vi "01 Dryer_Performance_SM.vi"() -> ()   [LabVIEW 2012] (continued)
      }
      frame "Data: Process RMC" {
        # "FIXME: RMC calculated after power on.  Is this OK?"
        # "Process Data Steps.\nPuts the gathered data into arrays to be saved."
        n763 = local read "Init Offset Coeff"() -> (w1636:dbl)
        n764 = local read "Offset"() -> (w1637:dbl)
        n765 = Unbundle By Name(w1689) -> ("Graph Reset"=w1686:bool, "Q Element"=w1684:T10, "Enable RMC"=w1651:bool)
        n766 = call "FGV Double.vi"() -> ("Value"=w1643:dbl)  [unwired: 11 in]
        n767 = Multiply(x=w1636, y=w1643) -> (x*y=w1642:dbl)
        n768 = Add(x=w1637, y=w1642) -> (x+y=w1641:dbl)
        "Load Offset" <- w1641
        n769 = Unbundle By Name(w1684) -> ("Label Array"=w1671:string[], "Data Array"=w1668:dbl[])
        n770 = Or(x=w1686, y="Clear Graph") -> (x .or. y?=w1683:bool)
        n771 = case shown="False" w1683 {
          tunnel: [w1707 w1710] -> w1682
          tunnel: "Plot: Add Data All\nPlot: Add Data Power\nPlot: Add Data RMC" ("State(s) in Front (\"\")") -> [w1709 w1710]
          frame True {
            n772 = Concatenate Strings("Plot: Init\n" ("State(s) in Front (\"\")"), w1709) -> (w1707:string)
          }
          frame False {
          }
        }
        n773 = local read "Wet Clothing Weight"() -> (w1679:dbl)
        n774 = for {
          tunnel: w1671 -> [w1706]
          tunnel: string[] ["Weight", "Room Ambient(F)", "RDB F", "Tscale"] -> [w1705] mode=indexing
          tunnel: w1668 -> [w1704]
          tunnel: [w1702] -> w1676 mode=indexing
          n775 = Search 1D Array(1D array=w1706, element=w1705) -> (index of element=w1703:i32)  [unwired: 1 in]
          n776 = Index Array(array=w1704, index=w1703) -> (element=w1702:dbl)
        }
        n777 = local read "Init Scale Temp"() -> (w1650:dbl)
        n778 = local read "Empty Dryer Cold Weight"() -> (w1680:dbl)
        n779 = local read "BDW - Bone Dry Wt(lbs)"() -> (w1681:dbl)
        n780 = Select(t=w1641, s="Apply Load Offset", f=0.0) -> (s? t:f=w1640:dbl)
        n781 = Array To Cluster(array=w1676) -> (cluster=w1675:T32)
        n782 = Unbundle(w1675) -> ("[0]"=w1655:dbl, "[1]"=w1667:dbl, "[2]"=w1666:dbl, "[3]"=w1660:dbl)
        "Scale (LBS)" <- w1655
        "Room Ambient F" <- w1667
        "RDB F" <- w1666
        n783 = Bundle(cluster=T7 {"Measeured Weight"=0.0, "BDW - Bone Dry Wt(lbs)"=0.0, "Empty Dryer Cold Weight"=0.0, "Measured IMC"=0.0, "Tamb"=0.0, "T-RDB"=0.0, "Drum Volume"=0.0, "Load Offset"=0.0, "Temp Coeff"=0.0, "Temp Cal"=0.0, "Tscale"=0.0} ("RMC Calc Inputs 2"), "Measeured Weight"=w1655, "BDW - Bone Dry Wt(lbs)"=w1681, "Empty Dryer Cold Weight"=w1680, "Measured IMC"=w1679, "Tamb"=w1667, "T-RDB"=w1666, "Drum Volume"="Drum Volume", "Load Offset"=w1640, "Temp Coeff"="Scale Temp Coeff", "Temp Cal"=w1650, "Tscale"=w1660) -> (w1673:T7)
        "RMC Calc Inputs" <- w1673
        n784 = local read "Power On One Shot"() -> (w1654:bool)
        n785 = local read "Use Smoothing"() -> (w1644:bool)
        n786 = case shown="True" w1654 {
          tunnel: w1673 -> [_ w1701]
          tunnel: [w1692 w1700] -> w1648
          tunnel: "MA Filter Size" -> [_ w1699]
          tunnel: [_ w1698] -> w1661
          tunnel: [w1692 w1697] -> w1658
          tunnel: [_ w1696] -> w1656
          tunnel: [_ w1695] -> w1652
          tunnel: w1651 -> [_ w1694]
          tunnel: [w1692 w1693] -> w1645
          frame False {
            w1692 = 0.0 ("RMC")
          }
          frame True {
            n787 = call "MA Scale Corrections.vi"("RMC Calc Inputs"=w1701, "Enable"=w1694, "MA Filter Size"=w1699) -> ("RMC_Sm"=w1693:dbl, "RMC"=w1700:dbl, "Raw Weight"=w1698:dbl, "Corrected Weight"=w1696:dbl, "Wcomp"=w1697:dbl, "Wbouy"=w1695:dbl)  [unwired: 11 in]
          }
        }
        "Cloth Weight(est.)" <- w1656
        "Wbouy" <- w1652
        n788 = Build Array (concatenate)(w1671, "Smooth_Rmc" ("element"), "RMC" ("element"), "Raw Weight" ("element"), "Corrected Weight" ("element"), "Wcomp" ("element"), "Wbouy" ("element")) -> (w1670:string[])
        n789 = call <vilib>:"Add State(s) to Queue__jki_lib_state_machine.vi"("State(s) in Front (\"\")"=w1682, "State(s) in (\"\")"=w1691) -> ("States Out"=w1690:string)  [unwired: 13 in]
        n790 = Select(t=w1645, s=w1644, f=w1648) -> (s? t:f=→"RMC%":dbl)
        n791 = Build Array(w1645, w1648, w1661, w1656, w1658, w1652) -> (w1663:dbl[])
        n792 = Build Array (concatenate)(w1668, w1663) -> (w1669:dbl[])
        n793 = Bundle By Name(cluster=w1689, "Graph Reset"=FALSE, "Q Element.Data Array"=w1669, "Q Element.Label Array"=w1670) -> (w1688:T29)
      }
      frame "Data: Save" {
        n794 = Unbundle By Name(w1716) -> ("Init Save File"=w1719:bool, "Q Element.Label Array"=w1717:string[], "Q Element.Data Array"=w1718:dbl[], "Q Element.Date"=w1713:string)
        n795 = local read "Write to File"() -> (w1720:bool)
        n796 = case shown="True" w1720 {
          tunnel: w1719 -> [w1724 w1733]
          tunnel: w1718 -> [_ w1732]
          tunnel: w1717 -> [_ w1731]
          tunnel: [w1724 FALSE ("Init Save File")] -> w1714
          tunnel: w1713 -> [_ w1728]
          tunnel: w1712 -> [w1723 w1726]
          tunnel: [w1723 w1725] -> w1711
          frame False {
          }
          frame True {
            n797 = Build Array("Date" ("delimiter (\\t)"), w1728) -> (w1727:string[])
            n798 = local read "FileName DataLog"() -> (w1734:path)
            n799 = case shown="False" w1733 {
              tunnel: w1734 -> [w1745 w1752]
              tunnel: w1732 -> [w1744 w1751]
              tunnel: w1731 -> [w1742 _]
              tunnel: w1727 -> [w1738 _]
              tunnel: w1726 -> [w1736 w1747]
              tunnel: [w1735 w1746] -> w1725
              frame True {
                n800 = Number To Fractional String(number=w1744) -> (F-format string=w1743:string[])  [unwired: 3 in]
                n801 = Build Array(w1742, w1743) -> (w1739:string[][])
                n802 = Build Array (concatenate)(w1738, w1739) -> (w1737:string[][])
                n803 = call "Write To Spreadsheet File (string) with Error.vi"("file path (dialog if empty)"=w1745, "2D data"=w1737, "append to file? (new file:F)"=TRUE, "error in"=w1736, "delimiter (\\t)"="," ("delimiter (\\t)")) -> ("error out"=w1735:errorcluster)  [unwired: 3 in, 1 out]
              }
              frame False {
                n804 = Number To Fractional String(number=w1751) -> (F-format string=w1748:string[])  [unwired: 3 in]
                n805 = call "Write To Spreadsheet File (string) with Error.vi"("file path (dialog if empty)"=w1752, "1D data"=w1748, "append to file? (new file:F)"=TRUE, "error in"=w1747, "delimiter (\\t)"="," ("delimiter (\\t)")) -> ("error out"=w1746:errorcluster)  [unwired: 3 in, 1 out]
              }
            }
          }
        }
        n806 = call <vilib>:"Add State(s) to Queue__jki_lib_state_machine.vi"("State(s) in (\"\")"=w1722) -> ("States Out"=w1721:string)  [unwired: 14 in]
        n807 = Bundle By Name(cluster=w1716, "Init Save File"=w1714) -> (w1715:T29)
      }
      frame "------PLOT-------" {
        # "Do not put any code in this frame.\n(It is a separator no-op. You can make a copy of this frame to create a new Data frame)"
        n808 = call <vilib>:"Add State(s) to Queue__jki_lib_state_machine.vi"("State(s) in (\"\")"=w1756) -> ("States Out"=w1755:string)  [unwired: 14 in]
      }
      frame "Plot: Init" {
        w1757 = cluster{dbl[], dbl[]}[] [] ("RHS Tank TCs")
        w1763 = TRUE  # Init Save File
        w1764 = FALSE  # Graph Reset
        # "Remove Time"
        n809 = Unbundle By Name(w1762) -> ("Q Element.Label Array"=w1761:string[])
        n810 = Delete From Array(array=w1761, length=1, index=0) -> (array with subset deleted=w1760:string[])  [unwired: 1 out]
        n811 = stacked-sequence {
          tunnel: w1760 -> [w1782 _ _]
          frame #0 {
            n812 = Array Size(array=w1782) -> (size(s)=w1781:i32)
            n813 = local read "Plot Legend"() -> (w1771:T2)
            n814 = local read "Number of TCs"() -> (w1780:i32)
            n815 = Index Array(array=w1771, index=0) -> (element=w1770:T30)
            n816 = To Unsigned Long Integer(number=w1781) -> (unsigned 32bit integer=w1783:u32)
            n817 = for {
              tunnel: w1782 -> [w1786] mode=indexing
              tunnel: w1780 -> [w1793]
              tunnel: w1770 -> [w1788]
              tunnel: [w1787] -> w1769 mode=indexing
              i -> [w1794]
              n818 = Less?(x=w1794, y=w1793) -> (x < y?=w1791:bool)
              n819 = Boolean To (0,1)(Boolean=w1791) -> (0, 1=w1792:i16)
              n820 = To Unsigned Long Integer(number=w1794) -> (unsigned 32bit integer=w1795:u32)
              n821 = property on="Plot All" class="XYGraph (strict)"("Active Plot"=w1795, "Plot.Plot Name"=w1786, "Plot.YScaleIdx"=w1792) -> ("Plot.Plot Color"=w1789:u32)  [unwired: 2 in, 2 out]
              n822 = Bundle By Name(cluster=w1788, "OnOff"=TRUE ("Boolean"), "Color Box"=w1789, "Title"=w1786) -> (w1787:T30)
            }
            n823 = property on="Plot All" class="XYGraph (strict)"("XScale.NameLbl.Text"="Time" ("X Scale.Name Label.Text"), "ActYScl"=1 ("Active Y Scale"), "YScale.NameLbl.Text"="Temperature °F" ("X Scale Label"), "YScale.Minimum"=50.0 ("Y Scale.Range:Minimum"), "YScale.Maximum"=200.0 ("Y Scale.Range:Maximum"), "ActYScl"=0 ("Active Y Scale"), "YScale.NameLbl.Text"="kWatts, lbs.,V,A" ("Y Scale Label Right"), "YScale.Minimum"=0.0 ("Ymin Right"), "YScale.Maximum"=250.0 ("Y Scale.Range:Maximum"), "LegNumRows"=w1783) -> ()  [unwired: 2 in, 2 out]
            n824 = local write "Plot Legend"(w1769) -> ()
          }
          frame #1 {
            w1805 = string[] ["Irms:Element 1", "Irms:Element 2", "P:Sigma"]
            n825 = control-ref of="Plot Power"() -> (w1796:refnum<vi>)
            n826 = for {
              tunnel: w1805 -> [w1816] mode=indexing
              tunnel: 2 ("y") -> [w1811]
              tunnel: w1796 -> [w1810]
              i -> [w1814]
              n827 = Greater Or Equal?(x=w1814, y=w1811) -> (x >= y?=w1812:bool)
              n828 = Boolean To (0,1)(Boolean=w1812) -> (0, 1=w1813:i16)
              n829 = To Unsigned Long Integer(number=w1814) -> (unsigned 32bit integer=w1815:u32)
              n830 = property on="Property Node" class="XYGraph (strict)"(reference=w1810, "Active Plot"=w1815, "Plot.Plot Name"=w1816, "Plot.YScaleIdx"=w1813) -> ()  [unwired: 1 in, 2 out]
            }
            n831 = Array Size(array=w1805) -> (size(s)=w1808:i32)
            n832 = To Unsigned Long Integer(number=w1808) -> (unsigned 32bit integer=w1806:u32)
            n833 = property on="Property Node" class="XYGraph (strict)"(reference=w1796, "XScale.NameLbl.Text"="Time" ("X Scale.Name Label.Text"), "ActYScl"=1 ("Active Y Scale"), "YScale.NameLbl.Text"="Watts" ("Y Scale.Name Label.Text"), "YScale.Minimum"=0.0 ("Y Scale.Range:Minimum"), "YScale.Maximum"=5000.0 ("Y Scale.Range:Maximum"), "ActYScl"=0 ("Active Y Scale"), "YScale.NameLbl.Text"="Current(Amps)" ("Y Scale.Name Label.Text"), "YScale.Minimum"=0.0 ("Y Scale.Range:Minimum"), "YScale.Maximum"=32.0 ("Y Scale.Range:Maximum"), "LegNumRows"=w1806) -> ()  [unwired: 1 in, 2 out]
          }
          frame #2 {
            w1824 = string[] ["RAW Weight", "RMC"]
            n834 = control-ref of="Plot RMC"() -> (w1817:refnum<vi>)
            n835 = Array Size(array=w1824) -> (size(s)=w1827:i32)
            n836 = for {
              tunnel: w1824 -> [w1834] mode=indexing
              tunnel: w1817 -> [w1829]
              i -> [w1832]
              n837 = Equal To 0?(x=w1832) -> (x = 0?=w1830:bool)
              n838 = Boolean To (0,1)(Boolean=w1830) -> (0, 1=w1831:i16)
              n839 = To Unsigned Long Integer(number=w1832) -> (unsigned 32bit integer=w1833:u32)
              n840 = property on="Property Node" class="XYGraph (strict)"(reference=w1829, "Active Plot"=w1833, "Plot.Plot Name"=w1834, "Plot.YScaleIdx"=w1831) -> ()  [unwired: 1 in, 2 out]
            }
            n841 = To Unsigned Long Integer(number=w1827) -> (unsigned 32bit integer=w1825:u32)
            n842 = property on="Property Node" class="XYGraph (strict)"(reference=w1817, "XScale.NameLbl.Text"="Time" ("X Scale.Name Label.Text"), "ActYScl"=1 ("Active Y Scale"), "YScale.NameLbl.Text"="LBS" ("Y Scale.Name Label.Text"), "AutoscaleDelay"=sgl 0.0 ("Autoscale Delay"), "ActYScl"=0 ("Active Y Scale"), "YScale.NameLbl.Text"="RMC" ("Y Scale.Name Label.Text"), "YScale.Minimum"=0.0 ("Y Scale.Range:Minimum"), "YScale.Maximum"=100.0 ("Y Scale.Range:Maximum"), "LegNumRows"=w1825) -> ()  [unwired: 1 in, 2 out]
          }
        }
        n843 = Bundle By Name(cluster=w1762, "Graph Reset"=w1764, "Init Save File"=w1763) -> (w1765:T29)
        n844 = local write "Plot All"(w1757) -> ()
        n845 = local write "Plot Power"(w1757) -> ()
        n846 = local write "Plot RMC"(w1757) -> ()
        n847 = call <vilib>:"Add State(s) to Queue__jki_lib_state_machine.vi"("State(s) in (\"\")"=w1768) -> ("States Out"=w1767:string)  [unwired: 14 in]
      }
      frame "Plot: Add Data All" {
        # "Add Current Sample to Data Array"
        # "First Element Assumed to be Time."
        n848 = Unbundle By Name(w1854) -> ("Time Array"=w1853:dbl[], "Q Element.Data Array"=w1848:dbl[], "Data Array"=w1856:dbl[][])
        n849 = case shown="True" "None" {
          selector: "None" -> [w1868 _]
          tunnel: "Plot Legend" -> [w1869 w1872]
          tunnel: [w1869 w1871] -> w1839
          tunnel: [w1868 w1870] -> w1836
          frame False {
          }
          frame True {
            n850 = for {
              tunnel: w1872 -> [w1875] mode=indexing
              tunnel: [w1874] -> w1871 mode=indexing
              tunnel: [w1873] -> w1870
              w1873 = FALSE ("OnOff")
              n851 = Bundle By Name(cluster=w1875, "OnOff"=w1873) -> (w1874:T30)
            }
          }
        }
        n852 = local write "None"(w1836) -> ()
        n853 = case shown="True" "All" {
          tunnel: w1839 -> [w1861 w1864]
          tunnel: [w1861 w1863] -> w1837
          tunnel: [FALSE ("OnOff") FALSE ("OnOff")] -> w1835
          frame False {
          }
          frame True {
            n854 = for {
              tunnel: w1864 -> [w1867] mode=indexing
              tunnel: [w1866] -> w1863 mode=indexing
              n855 = Bundle By Name(cluster=w1867, "OnOff"=TRUE) -> (w1866:T30)
            }
          }
        }
        n856 = Delete From Array(array=w1848, length=1, index=0) -> (deleted portion=w1846:dbl[], array with subset deleted=w1847:dbl[])
        n857 = Transpose 2D Array(2D array=w1856) -> (transposed array=w1851:dbl[][])
        n858 = Build Array (concatenate)(w1853, w1846) -> (w1849:dbl[])
        n859 = Build Array (concatenate)(w1851, w1847) -> (w1852:dbl[][])
        n860 = Transpose 2D Array(2D array=w1852) -> (transposed array=w1850:dbl[][])
        n861 = control-ref of="Plot All"() -> (w1842:refnum<vi>)
        n862 = local write "Plot Legend"(w1837) -> ()
        n863 = local write "All"(w1835) -> ()
        n864 = for {
          tunnel: w1849 -> [w1882]
          tunnel: [w1881] -> w1843 mode=indexing
          tunnel: w1850 -> [w1880] mode=indexing
          tunnel: w1842 -> [w1879]
          tunnel: w1837 -> [w1877] mode=indexing
          i -> [w1878]
          n865 = Unbundle By Name(w1877) -> ("OnOff"=w1876:bool)
          n866 = Bundle(w1882, w1880) -> (w1881:cluster{dbl[], dbl[]})  [unwired: 1 out]
          n867 = property on="Property Node" class="XYGraph (strict)"(reference=w1879, "Active Plot"=w1878, "Plot.Visible?"=w1876) -> ()  [unwired: 1 in, 2 out]
        }
        "Plot All" <- w1843
        n868 = call <vilib>:"Add State(s) to Queue__jki_lib_state_machine.vi"("State(s) in (\"\")"=w1859) -> ("States Out"=w1858:string)  [unwired: 14 in]
        n869 = Bundle By Name(cluster=w1854, "Time Array"=w1849, "Data Array"=w1850) -> (w1855:T29)
      }
      frame "Plot: Add Data Power" {
        n870 = Unbundle By Name(w1900) -> ("Q Element.Label Array"=w1899:string[], "Time Array"=w1901:dbl[], "Data Array"=w1891:dbl[][])
        n871 = for {
          tunnel: w1899 -> [w1908]
          tunnel: string[] ["Irms:Element 1", "Irms:Element 2", "P:Sigma"] -> [w1907] mode=indexing
          tunnel: [w1906] -> w1898 mode=indexing
          n872 = Search 1D Array(1D array=w1908, element=w1907) -> (index of element=w1906:i32)  [unwired: 1 in]
        }
        n873 = Index Array(array=w1898, index #1=0 ("index"), index #2=1 ("index"), index #3=2 ("index")) -> (element #1=w1894:i32, element #2=w1893:i32, element #3=w1892:i32)
        n874 = Decrement(x=w1893) -> (x-1=w1884:i32)
        n875 = Decrement(x=w1894) -> (x-1=w1885:i32)
        n876 = Decrement(x=w1892) -> (x-1=w1883:i32)
        n877 = Index Array(array=w1891, index (row)=w1885) -> (element=w1890:dbl[])  [unwired: 1 in]
        n878 = Index Array(array=w1891, index (row)=w1884) -> (element=w1889:dbl[])  [unwired: 1 in]
        n879 = Index Array(array=w1891, index (row)=w1883) -> (element=w1888:dbl[])  [unwired: 1 in]
        n880 = Build Array(w1890, w1889, w1888) -> (w1887:dbl[][])
        n881 = for {
          tunnel: w1901 -> [w1911]
          tunnel: [w1910] -> w1902 mode=indexing
          tunnel: w1887 -> [w1909] mode=indexing
          n882 = Bundle("Time Array"=w1911, w1909) -> (w1910:cluster{"Time Array":dbl[], dbl[]})  [unwired: 1 out]
        }
        "Plot Power" <- w1902
        n883 = call <vilib>:"Add State(s) to Queue__jki_lib_state_machine.vi"("State(s) in (\"\")"=w1905) -> ("States Out"=w1904:string)  [unwired: 14 in]
      }
      frame "Plot: Add Data RMC" {
        # "Is the dry time and exponential?"
        n884 = Unbundle By Name(w1942) -> ("Q Element.Label Array"=w1941:string[], "Time Array"=w1931:dbl[], "Data Array"=w1912:dbl[][])
        n885 = local read "Debug Mode"() -> (w1920:bool)
        n886 = Select(t="RMC", s=w1920, f="Smooth_Rmc") -> (s? t:f=w1917:string)
        n887 = Build Array("Weight", w1917) -> (w1916:string[])
        n888 = for {
          tunnel: w1941 -> [w1949]
          tunnel: w1916 -> [w1948] mode=indexing
          tunnel: [w1947] -> w1940 mode=indexing
          n889 = Search 1D Array(1D array=w1949, element=w1948) -> (index of element=w1947:i32)  [unwired: 1 in]
        }
        n890 = local read "BDW - Bone Dry Wt(lbs)"() -> (w1925:dbl)
        n891 = local read "RMC Limit"() -> (w1929:dbl)
        n892 = Index Array(array=w1940, index #1=0 ("index"), index #2=1 ("index"), index #3=2 ("index")) -> (element #1=w1937:i32, element #2=w1936:i32, element #3=w1914:i32)
        n893 = local read "Wet Clothing Weight"() -> (w1930:dbl)
        n894 = Decrement(x=w1936) -> (x-1=w1932:i32)
        n895 = Decrement(x=w1937) -> (x-1=w1933:i32)
        n896 = Decrement(x=w1914) -> (x-1=w1913:i32)
        n897 = Index Array(array=w1912, index (row)=w1933) -> (element=w1923:dbl[])  [unwired: 1 in]
        n898 = Index Array(array=w1912, index (row)=w1932) -> (element=w1935:dbl[])  [unwired: 1 in]
        n899 = Divide(x=w1929, y=100.0) -> (x/y=w1927:dbl)
        n900 = Index Array(array=w1912, index (row)=w1913) -> ()  [unwired: 1 in, 1 out]
        n901 = Multiply(x=w1925, y=w1927) -> (x*y=w1926:dbl)
        n902 = Build Array(w1923, w1935) -> (w1934:dbl[][])
        n903 = Add(x=w1925, y=w1926) -> (x+y=w1924:dbl)
        n904 = for {
          tunnel: w1931 -> [w1952]
          tunnel: [w1951] -> w1943 mode=indexing
          tunnel: w1934 -> [w1950] mode=indexing
          n905 = Bundle("Time Array"=w1952, w1950) -> (w1951:cluster{"Time Array":dbl[], dbl[]})  [unwired: 1 out]
        }
        "Plot RMC" <- w1943
        n906 = call "Estimate Exp Completion time.vi"("IMC Weight"=w1930, "Completion Weight"=w1924, "Time Values"=w1931, "Weight Values"=w1923) -> ("Completion Time Estimate"=→"Experimental Completion Time Estimate":dbl)  [unwired: 9 in, 2 out]
        n907 = call <vilib>:"Add State(s) to Queue__jki_lib_state_machine.vi"("State(s) in (\"\")"=w1946) -> ("States Out"=w1945:string)  [unwired: 14 in]
      }
      frame "-------FINALIZE------ " {
        n908 = call <vilib>:"Add State(s) to Queue__jki_lib_state_machine.vi"("State(s) in (\"\")"=w1956) -> ("States Out"=w1955:string)  [unwired: 14 in]
      }
      frame "Finalize Sequence" {
        n909 = local read "FileName DataLog"() -> (w1960:path)
        n910 = local read "Write to File"() -> (w1959:bool)
        n911 = call <vilib>:"Check if File or Folder Exists.vi"("path"=w1960) -> ("file or folder exists?"=w1958:bool)  [unwired: 8 in, 2 out]
        n912 = And(x=w1958, y=w1959) -> (x .and. y?=w1957:bool)
        n913 = case shown="True" w1957 {
          tunnel: [_ "Finalize DataLog\nFinalize Write DOE Data\nFinalize Move and Lock Files\nFinalize Zip Files" ("State(s) in Front (\"\")")] -> w1961
          frame False {
          }
          frame True {
          }
        }
        n914 = call <vilib>:"Add State(s) to Queue__jki_lib_state_machine.vi"("State(s) in Front (\"\")"=w1961, "State(s) in (\"\")"=w1965) -> ("States Out"=w1964:string)  [unwired: 13 in]
      }
      frame "Finalize DataLog" {
        w1971 = 60.0  # s/min
        # "RMC OK?"
        n915 = case shown="True" "Auto Scale Reading" {
          tunnel: [w2028 w2035] -> w2013
          tunnel: [w2026 w2033] -> w1974
          frame False {
            n916 = flat-sequence {
              tunnel: [w2030] -> w2027
              tunnel: [w2032] -> w2028
              tunnel: w2027 -> [w2032]
              tunnel: [w2031] -> w2026
              frame #0 {
                n917 = call "Panel Get Final Weight.vi"("Init value(\"\")"="0." ("Init value(\"\")")) -> ("Final Load  Weight Out"=w2030:string)  [unwired: 14 in]
              }
              frame #1 {
                n918 = call "E-Time.vi"() -> ("Elapsed Time (sec)"=w2031:dbl)  [unwired: 9 in, 2 out]
              }
            }
          }
          frame True {
            n919 = flat-sequence {
              tunnel: [w2037] -> w2034
              tunnel: [w2039] -> w2035
              tunnel: w2034 -> [w2039]
              tunnel: [w2038] -> w2033
              frame #0 {
                n920 = local read "Scale Com Port"() -> (w2036:refnum<visa-resource-name>)
                n921 = call "Panel Scale Reading Percision.vi"("VISA resource name"=w2036) -> ("read buffer"=w2037:string)  [unwired: 14 in]
              }
              frame #1 {
                n922 = call "E-Time.vi"() -> ("Elapsed Time (sec)"=w2038:dbl)  [unwired: 9 in, 2 out]
              }
            }
          }
        }
        n923 = Unbundle By Name(w2017) -> ("Q Element.Label Array"=w1987:string[], "Q Element.Data Array"=w1988:dbl[])
        n924 = local read "FileName DataLog"() -> (w1977:path)
        n925 = call "Log String to Spreadsheet.vi"("String"="Stopped", "error in (no error)"=w2018, "FileName"=w1977) -> ("error out"=w2015:errorcluster)  [unwired: 8 in]
        n926 = for {
          tunnel: w1987 -> [w2025]
          tunnel: string[] ["Time", "Gas Feedback", "Wp:Sigma"] -> [w2024] mode=indexing
          tunnel: w1988 -> [w2023]
          tunnel: [w2021] -> w1989 mode=indexing
          n927 = Search 1D Array(1D array=w2025, element=w2024) -> (index of element=w2022:i32)  [unwired: 1 in]
          n928 = Index Array(array=w2023, index=w2022) -> (element=w2021:dbl)
        }
        n929 = Fract/Exp String To Number(string=w2013) -> (number=w1991:dbl)  [unwired: 3 in, 1 out]
        n930 = local read "Use Dry Gas Meter?"() -> (w1984:bool)
        n931 = Concatenate Strings("Final Weight:, " ("String"), w2013) -> (w2007:string)
        n932 = local read "Enable RMC Limit"() -> (w1975:bool)
        n933 = local read "Power On One Shot"() -> (w2000:bool)
        n934 = call "Log String to Spreadsheet.vi"("String"=w2007, "error in (no error)"=w2015, "FileName"=w1977) -> ("error out"=w1979:errorcluster)  [unwired: 8 in]
        n935 = Array To Cluster(array=w1989) -> (cluster=w1990:cluster{"[0]":dbl, "[1]":dbl, "[2]":dbl})
        n936 = Unbundle(w1990) -> ("[0]"=w1973:dbl, "[1]"=w1981:dbl, "[2]"=w1980:dbl)
        n937 = Subtract(x=w1974, y=w1973) -> (x-y=w1972:dbl)
        n938 = Divide(x=w1972, y=w1971) -> (x/y=w1970:dbl)
        n939 = Number To Fractional String(number=w1970) -> (F-format string=w1969:string)  [unwired: 3 in]
        n940 = And(x=w1975, y=w2000) -> (x .and. y?=w2001:bool)
        n941 = Concatenate Strings("FMC DELAY (min):," ("String"), w1969) -> (w1968:string)
        n942 = call "Log String to Spreadsheet.vi"("String"=w1968, "error in (no error)"=w1979, "FileName"=w1977) -> ("error out"=w1978:errorcluster)  [unwired: 8 in]
        n943 = case shown="True" w2001 {
          tunnel: [TRUE w2041] -> w1999
          frame False {
          }
          frame True {
            n944 = local read "RMC Limit"() -> (w2042:dbl)
            n945 = local read "RMC%"() -> (w2043:dbl)
            n946 = Greater?(x=w2042, y=w2043) -> (0:w2041:bool)
          }
        }
        n947 = local read "BDW - Bone Dry Wt(lbs)"() -> (w2012:dbl)
        n948 = Select(t=w1981, s=w1984, f=0.0) -> (s? t:f=w1983:dbl)
        n949 = local read "End Msg"() -> (w2004:string)
        n950 = call "Log String to Spreadsheet.vi"("String"=w2004, "error in (no error)"=w1978, "FileName"=w1977) -> ()  [unwired: 8 in, 1 out]
        n951 = Divide(x=w1991, y=w2012) -> (x/y=w2011:dbl)
        n952 = call "Worksheet DOE Audit.vi"() -> ("DOE Data Out"=w1993:T23)  [unwired: 8 in, 2 out]
        n953 = Bundle By Name(cluster=w1993, "End Time(s)"=w1973, "Final Wt"=w1991, "Gas Vol Fin"=w1983, "Elect Energy End"=w1980) -> (w1992:T23)
        n954 = Decrement(x=w2011) -> (x-1=w2008:dbl)
        n955 = Search and Replace String(replace all?=TRUE ("replace all? (F)"), input string=w2004, search string=",") -> (result string=w2002:string)  [unwired: 5 in, 3 out]
        n956 = Number To Fractional String(number=w2008) -> (F-format string=w2010:string)  [unwired: 3 in]
        n957 = local read "2015?"() -> (w1967:bool)
        n958 = call "Worksheet DOE Audit.vi"("Add?"=TRUE, "DOE Data"=w1992, "2015?"=w1967) -> ()  [unwired: 5 in, 3 out]
        n959 = Concatenate Strings(w2002, "\r", "Final RMC:" ("String"), w2010) -> (w1998:string)
        n960 = call <vilib>:"Add State(s) to Queue__jki_lib_state_machine.vi"("State(s) in (\"\")"=w2020) -> ("States Out"=w2019:string)  [unwired: 14 in]
        n961 = Append True/False String(1:w1999, 2:". RMC Limit Not Reached." ("false string"), 3:"" ("true string"), 4:w1998) -> (0:→"Final User Message":string)
      }
      frame "Finalize Write DOE Data" {
        n962 = local read "FileName DataLog"() -> (w2045:path)
        n963 = call <vilib>:"Check if File or Folder Exists.vi"("path"=w2045) -> ("file or folder exists?"=w2046:bool)  [unwired: 8 in, 2 out]
        n964 = local read "2015?"() -> (w2044:bool)
        n965 = case shown="True" w2046 {
          tunnel: w2045 -> [_ w2052]
          tunnel: w2044 -> [_ w2051]
          frame False {
          }
          frame True {
            n966 = case shown="True" w2051 {
              tunnel: w2052 -> [w2063 w2069]
              frame False {
                n967 = Strip Path(path=w2063) -> (name=w2059:string)  [unwired: 1 out]
                n968 = Search and Replace String(input string=w2059, search string=".tmp", replace string="_OUT.txt" ("replace string (\"\")")) -> (result string=w2061:string)  [unwired: 5 in, 3 out]
                n969 = global read "Global Test Variables DPT.vi" "Globals for Dryer Performance Test"() -> (w2058:T9)
                n970 = Unbundle By Name(w2058) -> ("Directories.Data Backup Directory"=w2057:path)
                n971 = local read "2015?"() -> (w2055:bool)
                n972 = call "Worksheet DOE Audit.vi"("Write Form"=TRUE ("Add?"), "2015?"=w2055) -> ("String"=w2053:string)  [unwired: 6 in, 2 out]
                n973 = Build Path(base path=w2057, name or relative path=w2061) -> (appended path=w2054:path)
                "DOE Filename" <- w2054
                n974 = call "File Write with Filename.vi"("Path"=w2054, "text"=w2053) -> ()  [unwired: 12 in, 2 out]
                n975 = One Button Dialog(message=w2053) -> ()  [unwired: 1 in, 1 out]
              }
              frame True {
                n976 = Strip Path(path=w2069) -> (name=w2074:string)  [unwired: 1 out]
                n977 = Search and Replace String(input string=w2074, search string=".tmp", replace string="_OUT.csv" ("replace string (\"\")")) -> (result string=w2076:string)  [unwired: 5 in, 3 out]
                n978 = global read "Global Test Variables DPT.vi" "Globals for Dryer Performance Test"() -> (w2073:T9)
                n979 = Unbundle By Name(w2073) -> ("Directories.Data Backup Directory"=w2072:path)
                n980 = local read "Low Power Switch"() -> (w2065:bool)
                n981 = local read "2015?"() -> (w2070:bool)
                n982 = call "Worksheet DOE Audit.vi"("Write Form"=TRUE ("Add?"), "Low Power\nSwitch"=w2065, "2015?"=w2070) -> ("String"=w2064:string, "2015 array"=w2066:string[][])  [unwired: 5 in, 1 out]
                n983 = Build Path(base path=w2072, name or relative path=w2076) -> (appended path=w2068:path)
                n984 = local write "DOE Filename"(w2068) -> ()
                n985 = call-poly <vilib>:"Write To Spreadsheet File.vi"("delimiter (\\t)"="," ("delimiter (\\t)"), "2D data"=w2066, "file path (dialog if empty)"=w2068) -> ()  [unwired: 5 in, 1 out]
                n986 = One Button Dialog(message=w2064) -> ()  [unwired: 1 in, 1 out]
              }
            }
          }
        }
        n987 = call <vilib>:"Add State(s) to Queue__jki_lib_state_machine.vi"("State(s) in (\"\")"=w2050) -> ("States Out"=w2049:string)  [unwired: 14 in]
      }
      frame "Finalize Move and Lock Files" {
        n988 = local read "FileName DataLog"() -> (w2078:path)
        n989 = stacked-sequence {
          tunnel: w2078 -> [w2086 _ _ w2120]
          frame #0 {
            # "DC Voltages"
            n990 = Strip Path(path=w2086) -> (name=w2084:string)  [unwired: 1 out]
            n991 = Match Pattern(string=w2084, regular expression=".tmp" ("search string")) -> (before substring=→"Filename Prefix String":string)  [unwired: 1 in, 3 out]
          }
          frame #1 {
            # "DC Voltages"
            n992 = local read "Stream DC to File?"() -> (w2087:bool)
            n993 = case shown="True" w2087 {
              frame False {
              }
              frame True {
                n994 = global read "Global Test Variables DPT.vi" "Globals for Dryer Performance Test"() -> (w2096:T9)
                n995 = local read "Filename Prefix String"() -> (w2089:string)
                n996 = Unbundle By Name(w2096) -> ("Directories.Data Backup Directory"=w2095:path)
                n997 = local read "DC Voltages Filename"() -> (w2093:path)
                n998 = Concatenate Strings(w2089, "_DC_VOLTAGES.csv" ("search string")) -> (w2088:string)
                n999 = Build Path(base path=w2095, name or relative path=w2088) -> (appended path=w2092:path)
                n1000 = Copy(10:w2092, 11:w2093) -> (3:w2091:path)  [unwired: 3 in, 2 out]
                n1001 = local write "DC Voltages Filename"(w2091) -> ()
                n1002 = Set Permissions(7:i16 0 ("permissions"), 11:w2091) -> (0:w2097:errorcluster)  [unwired: 3 in, 1 out]
                n1003 = Merge Errors(w2097) -> ()  [unwired: 1 out]
              }
            }
          }
          frame #2 {
            n1004 = local read "Nufi?"() -> (w2098:bool)
            n1005 = case shown="False" w2098 {
              frame False {
              }
              frame True {
                n1006 = global read "Global Test Variables DPT.vi" "Globals for Dryer Performance Test"() -> (w2107:T9)
                n1007 = while {
                  tunnel: [w2111] -> w2105
                  stop <- w2111 stop-if-true
                  n1008 = local read "End4_Nufi"() -> (w2111:bool)
                  n1009 = case shown="False" w2111 {
                    frame False {
                      n1010 = Wait (ms)(milliseconds to wait=u32 250) -> ()  [unwired: 1 out]
                    }
                    frame True {
                    }
                  }
                }
                n1011 = local read "Filename Prefix String"() -> (w2100:string)
                n1012 = Unbundle By Name(w2107) -> ("Directories.Data Backup Directory"=w2106:path)
                n1013 = Concatenate Strings(w2100, "_NUFI_DEBUG.csv" ("search string")) -> (w2099:string)
                n1014 = flat-sequence {
                  tunnel: [w2110] -> w2103
                  tunnel: w2105 -> [_]
                  frame #0 {
                    n1015 = local read "Nufi Data File Path"() -> (w2110:path)
                  }
                }
                n1016 = Build Path(base path=w2106, name or relative path=w2099) -> (appended path=w2104:path)
                n1017 = Copy(10:w2104, 11:w2103) -> (3:w2102:path)  [unwired: 3 in, 2 out]
                n1018 = Set Permissions(7:i16 0 ("permissions"), 11:w2102) -> (0:w2108:errorcluster)  [unwired: 3 in, 1 out]
                n1019 = local write "Nufi Data File Path"(w2102) -> ()
                n1020 = Merge Errors(w2108) -> ()  [unwired: 1 out]
              }
            }
          }
          frame #3 {
            # "DATA LOG"
            n1021 = global read "Global Test Variables DPT.vi" "Globals for Dryer Performance Test"() -> (w2117:T9)
            n1022 = local read "Filename Prefix String"() -> (w2114:string)
            n1023 = Unbundle By Name(w2117) -> ("Directories.Data Backup Directory"=w2116:path)
            n1024 = Concatenate Strings(w2114, ".csv" ("search string")) -> (w2113:string)
            n1025 = Build Path(base path=w2116, name or relative path=w2113) -> (appended path=w2119:path)
            n1026 = Copy(10:w2119, 11:w2120) -> (3:w2118:path)  [unwired: 3 in, 2 out]
            n1027 = local write "FileName DataLog"(w2118) -> ()
          }
        }
        n1028 = call <vilib>:"Add State(s) to Queue__jki_lib_state_machine.vi"("State(s) in (\"\")"=w2082) -> ("States Out"=w2081:string)  [unwired: 14 in]
      }
      frame "Finalize Zip Files" {
        n1029 = local read "FileName DataLog"() -> (w2127:path)
        n1030 = global read "Global Test Variables DPT.vi" "Globals for Dryer Performance Test"() -> (w2149:T9)
        n1031 = while {
          tunnel: [w2156] -> w2123
          stop <- w2157 stop-if-true
          n1032 = local read "Nufi Data File Path"() -> (w2156:path)
          n1033 = local read "End4_Nufi"() -> (w2157:bool)
          n1034 = Wait (ms)(milliseconds to wait=u32 150) -> ()  [unwired: 1 out]
        }
        n1035 = local read "Stream DC to File?"() -> (w2150:bool)
        n1036 = Unbundle By Name(w2149) -> ("Directories.Save File Directory"=w2148:path, "Directories.Library Directory"=w2135:path, "Directories.Data Backup Dir Fail"=w2134:path, "Directories.Lab Directory"=w2133:path)
        n1037 = call <vilib>:"Three Button Dialog.vi"("Allow user to close window? (TRUE)"=FALSE, "Right Button Text (\"Cancel\")"="Lab Eval" ("Right Button Text (\"Cancel\")"), "Center Button Text (\"No\")"="Fail" ("F button name (\"Cancel\")"), "Left Button Text (\"Yes\")"="Pass" ("T button name (\"OK\")"), "message"="Final Test Result.  \"Pass\" will log data to the backup server.  \"Fail\" will copy files to another location.") -> ("Which Button?"=w2137:T33)  [unwired: 6 in]
        n1038 = case shown="True" w2150 {
          tunnel: [_ w2186] -> w2126
          frame False {
          }
          frame True {
            n1039 = local read "DC Voltages Filename"() -> (w2186:path)
          }
        }
        n1040 = case shown="\"Center Button\"" w2137 {
          tunnel: [w2175 w2180 w2185] -> w2136
          tunnel: w2135 -> [w2175 _ _]
          tunnel: w2134 -> [_ w2180 _]
          tunnel: w2133 -> [_ _ w2185]
          tunnel: ["Result: Pass" ("T button name (\"OK\")") w2177 w2182] -> w2132
          tunnel: [TRUE FALSE FALSE] -> w2128
          frame "Left Button", Default {
          }
          frame "Center Button" {
            n1041 = call "Prompt User for Input"() -> ("Reason for Failure"=w2178:string)  [unwired: 17 in, 2 out]
            n1042 = Concatenate Strings("Result: Fail - ", w2178) -> (w2177:string)
          }
          frame "Right Button" {
            n1043 = call "Prompt User for Input2"() -> ("Eval Description"=w2183:string)  [unwired: 17 in, 2 out]
            n1044 = Concatenate Strings("Result:  Eval -", w2183) -> (w2182:string)
          }
        }
        n1045 = call "Log String to Spreadsheet.vi"("String"=w2132, "error in (no error)"=w2124, "FileName"=w2127) -> ("error out"=w2130:errorcluster)  [unwired: 8 in]
        n1046 = local read "Filename Prefix String"() -> (w2145:string)
        n1047 = Set Permissions(7:i16 0 ("permissions"), 8:w2130, 11:w2127) -> (0:w2122:errorcluster)  [unwired: 2 in, 1 out]
        n1048 = case shown="False" w2128 {
          tunnel: w2127 -> [w2164 w2169]
          tunnel: w2126 -> [w2165 w2171]
          tunnel: w2123 -> [w2160 w2170]
          tunnel: [w2162 w2168] -> w2125
          tunnel: w2122 -> [w2159 w2167]
          tunnel: [w2158 w2167] -> w2121
          frame True {
            n1049 = call <vilib>:"Check if File or Folder Exists.vi"("path"=w2160) -> ("file or folder exists?"=w2161:bool)  [unwired: 8 in, 2 out]
            n1050 = local read "DOE Filename"() -> (w2166:path)
            n1051 = call "Parser Dryer Performance.vi"("error in"=w2159, "Process Debug?"=w2161, "log file path in"=w2164, "debug log path in"=w2160) -> ("error out"=w2158:errorcluster, "new file path out"=w2163:path)  [unwired: 6 in]
            n1052 = Build Array(w2166, w2164, w2165, w2160, w2163) -> (w2162:path[])
          }
          frame False {
            n1053 = local read "DOE Filename"() -> (w2172:path)
            n1054 = Build Array(w2172, w2169, w2171, w2170) -> (w2168:path[])
          }
        }
        n1055 = Concatenate Strings(w2145, "_OUT.zip" ("replace string (\"\")")) -> (w2144:string)
        n1056 = Build Path(base path=w2148, name or relative path=w2144) -> (appended path=w2143:path)
        "zip path" <- w2143
        n1057 = call <vilib>:"Add State(s) to Queue__jki_lib_state_machine.vi"("State(s) in (\"\")"=w2154) -> ("States Out"=w2153:string)  [unwired: 14 in]
        n1058 = call "Zip Array of Files.vi"("error in (no error)"=w2121, "Target Zip Filename"=w2143, "Files to Zip"=w2125) -> ("error out"=w2147:errorcluster)  [unwired: 8 in]
        n1059 = Copy(8:w2147, 10:w2136, 11:w2143) -> (0:w2129:errorcluster)  [unwired: 2 in, 2 out]
      }
      frame "Exit" {
        n1060 = call <vilib>:"Add State(s) to Queue__jki_lib_state_machine.vi"("State(s) in (\"\")"=w2191) -> ("States Out"=w2190:string)  [unwired: 14 in]
      }
    }
    n1061 = local read "Debug Mode"() -> (w1422:bool)
    n1062 = case shown="True" w1422 {
      tunnel: w1425 -> [w1435 w1438]
      tunnel: [w1435 w1437] -> w1424
      tunnel: w1423 -> [_ w1436]
      frame False {
      }
      frame True {
        n1063 = Build Array (concatenate)(w1438, w1436) -> (w1437:string[])
        "UI States" <- w1437
      }
    }
  }
  n1064 = while "Data Acquisition Steps" {
    shift-right: [w2203] -> _
    shift-left: _ -> [w2202]
    shift-right: [w2205] -> _
    shift-left: _ -> [w2201]
    shift-right: [w2204] -> _
    shift-left: w14 -> [w2206]
    shift-right: [w2200] -> w9
    shift-left: 0.0 ("Elapsed Time (sec)") -> [w2199]
    tunnel: w23 -> [w2192]
    shift-right: [w2198] -> _
    shift-left: string[] [] -> [w2197]
    tunnel: [w2193] -> w8
    tunnel: [w2192] -> w11
    stop <- w2193 stop-if-true
    # "Data Log Time"
    n1065 = call <vilib>:"Parse State Queue__jki_lib_state_machine.vi"("State Queue"=w2206, "Error In (no error)"=w2201) -> ("Remaining States"=w2208:string, "Current State"=w2196:string, "Arguments"=w2207:string)  [unwired: 11 in]
    n1066 = case shown="\"Data Acquire: CDAQ\"" w2196 {
      selector: w2196 -> [_ w2246 _ _ _ _ _ w2328 w2380 w2466 w2527 w2562 w2596 _ _]
      tunnel: w2208 -> [w2223 w2250 w2267 w2273 w2278 w2285 w2314 w2331 w2383 w2469 w2538 w2571 w2601 w2653 w2687]
      tunnel: w2207 -> [_ _ _ _ _ _ _ _ _ _ _ _ _ _ _]
      tunnel: w2202 -> [w2221 w2248 w2260 w2271 w2275 _ w2309 w2334 w2384 w2471 w2534 w2567 w2597 w2649 w2681]
      tunnel: [w2220 w2252 errorcluster {"status"=FALSE, "code"=0, "source"=""} ("error out") w2268 w2276 w2283 w2312 w2329 w2381 w2467 w2521 w2559 w2594 w2647 w2685] -> w2205
      tunnel: w2201 -> [w2219 w2251 w2258 w2268 w2276 w2283 w2312 w2335 w2385 w2472 w2530 w2560 w2595 w2648 w2685]
      tunnel: [w2222 w2249 w2266 w2272 w2277 w2284 w2317 w2338 w2388 w2475 w2537 w2570 w2600 w2652 w2686] -> w2204
      tunnel: [_ _ _ TRUE _ w2279 _ _ _ _ _ _ _ _ _] -> w2193
      tunnel: [w2218 w2248 w2260 w2271 w2275 w2281 w2315 w2336 w2386 w2473 w2535 w2568 w2598 w2650 w2681] -> w2203
      tunnel: "DAQ Timer" -> [w2217 _ _ _ _ _ _ _ _ _ _ _ _ _ _]
      tunnel: [w2215 w2245 w2263 w2270 w2274 w2282 w2316 w2337 w2387 w2474 w2536 w2569 w2599 w2651 w2682] -> w2200
      tunnel: w2199 -> [w2214 w2245 w2263 w2270 w2274 w2282 w2316 w2337 w2387 w2474 w2536 w2569 w2599 w2651 w2682]
      tunnel: w2192 -> [_ _ _ _ _ w2280 _ _ _ _ _ _ _ _ w2679]
      frame "", "Idle" {
        n1067 = call "E-Time.vi"() -> ("Elapsed Time (sec)"=w2213:dbl)  [unwired: 9 in, 2 out]
        n1068 = call "Timeout Calc.vi"("Complete time"=w2213, "Gather Data Period"=w2217, "Start Time"=w2214) -> ("Delay Time"=w2216:i32)  [unwired: 8 in]
        "DAQ Delay Time" <- w2216
        n1069 = event shown="[0] Timeout;  \"Get Data Interrupt\": Value Change" {
          selector: _ -> [_]
          dyn-events: _ -> [_]
          timeout: w2216 -> [_]
          tunnel: w2223 -> [w2233]
          tunnel: [w2232] -> w2222
          tunnel: w2221 -> [w2230]
          tunnel: [w2231] -> w2220
          tunnel: w2219 -> [w2231]
          tunnel: [w2230] -> w2218
          tunnel: [w2227] -> w2215
          event Timeout; "Get Data Interrupt": Value Change {
            # "Edit Data Acquisition Steps.\n(These are the steps used to gather the data.)"
            n1070 = event-data() -> ()  [unwired: 1 in, 1 out]
            n1071 = call "E-Time.vi"() -> ("Elapsed Time (sec)"=w2227:dbl)  [unwired: 9 in, 2 out]
            n1072 = local read "Loggin Data"() -> (w2229:bool)
            n1073 = local read "cDAQ"() -> (w2224:bool)
            n1074 = case shown="True" w2224 {
              tunnel: [w2234 w2235] -> w2226
              frame True {
                w2234 = "Data Acquire: Init\nData Acquire: CDAQ\nData Acquire: Power\nData Acquire: Gas\nData Acquire: RH\nData: Queue"  # Data Acquisition Steps
              }
              frame False {
                w2235 = "Data Acquire: Init\nData Acquire: Ag + W\nData Acquire: Power\nData Acquire: Gas\nData Acquire: RH\nData: Queue"  # Data Acquisition Steps
              }
            }
            n1075 = case shown="False" w2229 {
              tunnel: [w2237 w2242] -> w2228
              tunnel: w2227 -> [_ _]
              tunnel: w2226 -> [_ w2240]
              frame False {
                n1076 = local read "End1_Main"() -> (w2236:bool)
                n1077 = case shown="True" w2236 {
                  tunnel: ["" " Exit"] -> w2237
                  frame False {
                  }
                  frame True {
                  }
                }
              }
              frame True {
                n1078 = local read "End1_Main"() -> (w2241:bool)
                n1079 = case shown="True" w2241 {
                  tunnel: [w2243 "Exit"] -> w2242
                  tunnel: w2240 -> [w2243 _]
                  frame False {
                  }
                  frame True {
                  }
                }
              }
            }
            n1080 = local write "Get Data Interrupt"(FALSE ("Get Data Interrupt")) -> ()
            n1081 = call <vilib>:"Add State(s) to Queue__jki_lib_state_machine.vi"("State(s) in Front (\"\")"=w2228, "State(s) in (\"\")"=w2233) -> ("States Out"=w2232:string)  [unwired: 13 in]
          }
        }
      }
      frame Default {
        w2255 = 42 items=["No error", "Argument error", "Memory is full", "Out of zone", "End of file", "File already open", "Generic file I/O error", "File not found", "File permission error", "Disk is full", "Duplicate path", "Too many files open", "System feature not enabled", "Resource file not found", "Cannot add resource", "Resource not found", "Image not found", "Image memory error", "Pen does not exist", "Config type invalid", "Config token not found", "Config parse error", "Config memory error", "Bad external code format", "Bad external code offset", "External code not present", "Null window", "Destroy window error", "Null menu", "Print aborted", "Bad print record", "Print driver error", "Windows error during printing", "Memory error during printing", "Print dialog error", "Generic print error", "Invalid device refnum", "Device not found", "Device parameter error", "Device unit error", "Cannot open device", "Device call aborted", "Generic error", "Cancelled by user", "Object ID too low", "Object ID too high", "Object not in heap", "Unknown heap", "Unknown object (invalid DefProc)", "Unknown object (DefProc not in table)", "Message out of range", "Invalid (null) method", "Unknown message", "Manager call not supported", "Bad address", "Network operation in progress", "Network operation timed out", "Connection is busy", "Network attribute not supported", "Network error", "Address in use", "System out of memory", "Connection aborted", "Connection refused", "Not connected", "Already connected", "Connection closed", "Initialization error (interapplication manager)", "Bad occurrence", "Wait on unbound occurrence handler", "Occurrence queue overflow", "Datalog type conflict", "Unused", "Unrecognized type (interapplication manager)", "Memory corrupt", "Failed to make temporary DLL", "Old CIN version", "Drag socket not found", "Failed to load drop-object", "Failed to register OLE object", "Failed to release OLE object", "Format specifier type mismatch", "Unknown format specifier", "Too few format specifiers", "Too many format specifiers", "Scan failed", "Newer CIN version", "Error converting to variant", "Runtime menu error", "Password tampered", "Variant attribute not found", "Incompatible variant data type", "Event data is not available", "Event Store is not present", "Occurrence is not found", "Event Queue is not created", "Event info is not available", "Refnum passed is NULL", "Error retrieving Class GUID", "Error retrieving CoClass GUID", "Error retrieving TypeLib GUID.", "Bad built application magic bytes.", "Specific driver is different from the specific driver associated with the Logical Name.", "There is no session opened to the class driver.", "Max Error", "MAX - Error with config objects", "MAX - Error loading configuration", "MAX - Group not supported"]
        # "Current State"
        # "Do not delete, rename, or modify this frame.\n(this is used to capture unhandled states and typos)"
        # "Handle mistyped state name (developer tool)"
        n1082 = Format Into String(format string="Software Exception: Unhandled State \"%s\"." ("message"), error in=w2251, w2246) -> (resulting string=w2254:string, error out=w2253:errorcluster)  [unwired: 1 in]
        n1083 = call <vilib>:"Error Cluster From Error Code.vi"("show call chain? (False)"=TRUE, "error in (no error)"=w2253, "error message (\"\")"=w2254, "error code (0)"=w2255) -> ("error out"=w2252:errorcluster)  [unwired: 5 in]
        n1084 = call <vilib>:"Add State(s) to Queue__jki_lib_state_machine.vi"("State(s) in (\"\")"=w2250) -> ("States Out"=w2249:string)  [unwired: 14 in]
      }
      frame "Error Handler" {
        # "Unhandled Error -- Display it"
        # "Handle any errors here.\nYou can also output any states to clean-up after errors occur"
        # "Clear error"
        n1085 = Unbundle By Name(w2260) -> ("Error Log 2"=w2259:errorcluster[])
        n1086 = call <vilib>:"General Error Handler.vi"("error in (no error)"=w2258) -> ()  [unwired: 10 in, 5 out]
        n1087 = Build Array (concatenate)(w2259, w2258) -> (w2257:errorcluster[])
        n1088 = Bundle By Name(cluster=w2260, "Error Log 2"=w2257) -> ()  [unwired: 1 out]
        n1089 = control-ref of="This VI"() -> (w2262:refnum<vi>)
        n1090 = local write "Error Log 2"(w2257) -> ()
        n1091 = property class="VI"(reference=w2262, "TB.ShowAbortBut"=TRUE ("Tool Bar:Show Abort Button")) -> ()  [unwired: 1 in, 2 out]
        n1092 = call <vilib>:"Add State(s) to Queue__jki_lib_state_machine.vi"("State(s) in Front (\"\")"="/* Post Error States", "State(s) in (\"\")"=w2267) -> ("States Out"=w2266:string)  [unwired: 13 in]
      }
      frame "Exit" {
        n1093 = call <vilib>:"Add State(s) to Queue__jki_lib_state_machine.vi"("State(s) in (\"\")"=w2273) -> ("States Out"=w2272:string)  [unwired: 14 in]
      }
      frame "---------- Data ----------" {
        # "Do not put any code in this frame.\n(It is a separator no-op. You can make a copy of this frame to create a new Data frame)"
        n1094 = call <vilib>:"Add State(s) to Queue__jki_lib_state_machine.vi"("State(s) in (\"\")"=w2278) -> ("States Out"=w2277:string)  [unwired: 14 in]
      }
      frame "Data: Initialize" {
        # "Initialize Data.\n(This is the initialization of all of the data to be Logged.)"
        n1095 = while {
          tunnel: [w2297] -> w2281
          tunnel: w2280 -> [w2296]
          tunnel: [w2289] -> w2279
          stop <- w2290 continue-if-true
          w2293 = T10 {"Data Array"=[], "Label Array"=[], "Date"=""}  # Q Element
          w2294 = dbl[] []  # Data Array
          # "Wait till init complete, or finish."
          n1096 = Wait (ms)(milliseconds to wait=u32 150) -> ()  [unwired: 1 out]
          n1097 = local read "DAQ Chanel List"() -> (w2287:string)
          n1098 = local read "Equipment"() -> (w2295:T6)
          n1099 = Bundle(cluster=w2293, "Data Array"=w2294) -> (w2292:T10)  [unwired: 2 in]
          n1100 = Bundle("queue out"=w2296, "Q Element"=w2292, "Equipment"=w2295, "DAQ Chanel List"=w2287, "Error Log 2"="Error Log 2") -> (w2297:T34)  [unwired: 1 in]
          n1101 = local read "Loggin Data"() -> (w2291:bool)
          n1102 = local read "End1_Main"() -> (w2289:bool)
          n1103 = Compound Arithmetic op=AND(invert w2289, invert w2291) -> (w2290:bool)
        }
        n1104 = call <vilib>:"Add State(s) to Queue__jki_lib_state_machine.vi"("State(s) in (\"\")"=w2285) -> ("States Out"=w2284:string)  [unwired: 14 in]
      }
      frame "Data Acquire: Init" {
        # "On all of the data, we have a label in the label array, and the data in the Data array."
        # "Acquire Data Step.\n(This is an example that simulates the gathering of data.)"
        n1105 = Unbundle By Name(w2309) -> ("Q Element.Data Array"=w2308:dbl[])
        n1106 = Index Array(array=w2308, index=0) -> (element=w2305:dbl)
        n1107 = call "E-Time.vi"() -> ("Elapsed Time (sec)"=w2306:dbl)  [unwired: 9 in, 2 out]
        n1108 = Get Date/Time String(want seconds? (F)=TRUE) -> (date string=w2299:string, time string=w2300:string)  [unwired: 2 in]
        n1109 = Subtract(x=w2306, y=w2305) -> (x-y=→"Tsamp(s)":dbl)
        n1110 = local read "DAQ Chanel List"() -> (w2303:string)
        n1111 = Concatenate Strings(w2299, ", " ("string"), w2300) -> (w2298:string)
        n1112 = Build Array(w2306) -> (w2313:dbl[])
        n1113 = Build Array("Time") -> (w2310:string[])
        n1114 = Bundle By Name(cluster=w2309, "DAQ Chanel List"=w2303, "Q Element.Label Array"=w2310, "Q Element.Data Array"=w2313, "Q Element.Date"=w2298) -> (w2315:T34)
        n1115 = call <vilib>:"Add State(s) to Queue__jki_lib_state_machine.vi"("State(s) in (\"\")"=w2314) -> ("States Out"=w2317:string)  [unwired: 14 in]
      }
      frame "Data Acquire: Agilent" {
        # "First one begins array."
        # "Acquire Data Step.\n(This is an example that simulates the gathering of data.)"
        n1116 = Unbundle By Name(w2334) -> ("Q Element.Label Array"=w2325:string[], "Q Element.Data Array"=w2324:dbl[], "Equipment.Com Agilent"=w2333:refnum<visa-resource-name>)
        n1117 = local read "Simulate"() -> (w2330:bool)
        n1118 = local read "DAQ Label List"() -> (w2318:string[])
        n1119 = case shown="False" w2330 {
          tunnel: w2335 -> [w2353 w2360]
          tunnel: w2333 -> [w2352 _]
          tunnel: [w2349 w2356] -> w2323
          tunnel: [w2348 "Simulation" ("Error Message")] -> w2332
          tunnel: [w2347 w2360] -> w2329
          tunnel: w2318 -> [_ w2358]
          frame False {
            n1120 = call "AG34980A Initiate.vi"("VISA resource name"=w2352, "error in (no error)"=w2353) -> ("VISA resource name out"=w2351:refnum<visa-resource-name>, "error out"=w2355:errorcluster)  [unwired: 12 in]
            n1121 = call "AG34980A Fetch.vi"("VISA resource name"=w2351, "Numbers Only (T:On)"=TRUE, "error in (no error)"=w2355) -> ("VISA resource name out"=w2350:refnum<visa-resource-name>, "Output Data (Numbers Only)"=w2349:dbl[], "error out"=w2354:errorcluster)  [unwired: 8 in, 2 out]
            n1122 = call "AG34980A Error Query (Multiple).vi"("VISA resource name"=w2350, "error in (no error)"=w2354) -> ("Error Message"=w2348:string, "error out"=w2347:errorcluster)  [unwired: 10 in, 2 out]